vi "Visualizacion_NEW.vi"() -> ()   [LabVIEW 2021] (continued)
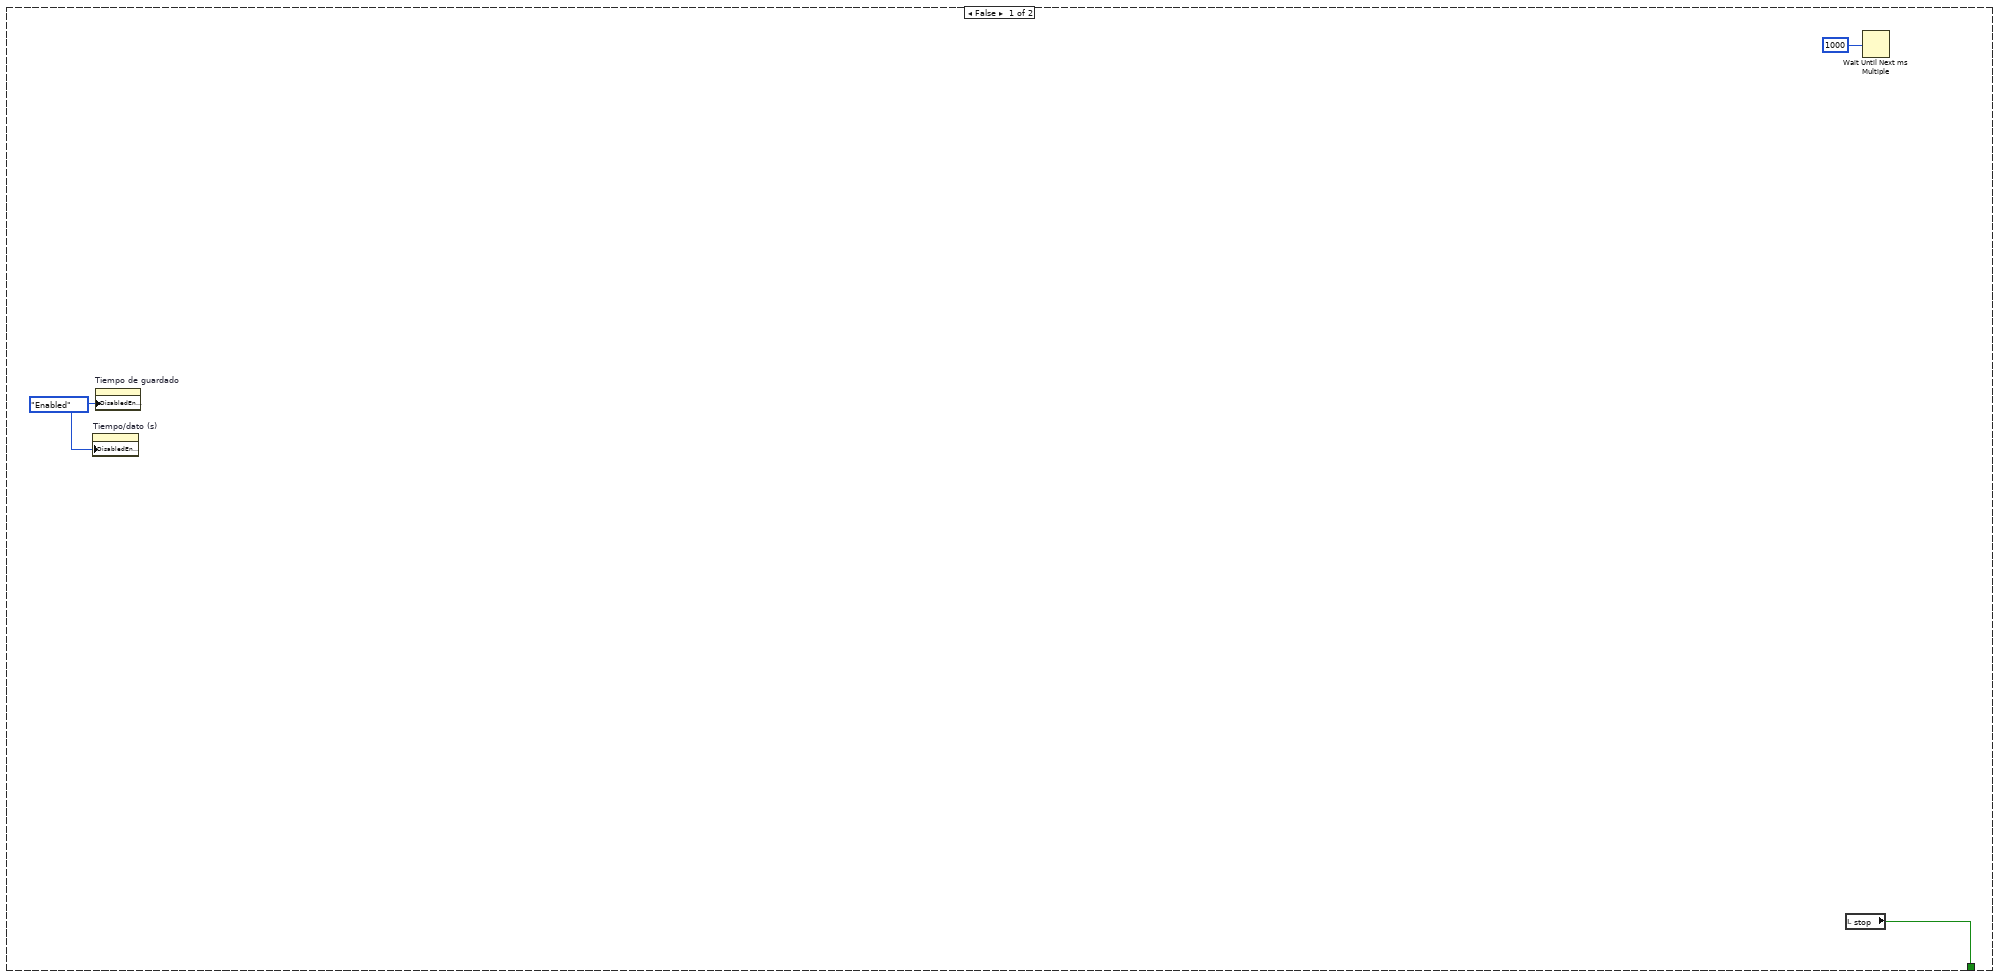
[diagram p2: hidden frame]
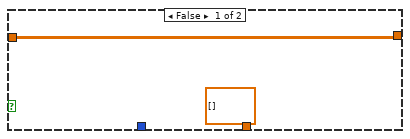
[diagram p3: hidden frame]
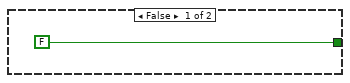
[diagram p4: hidden frame]
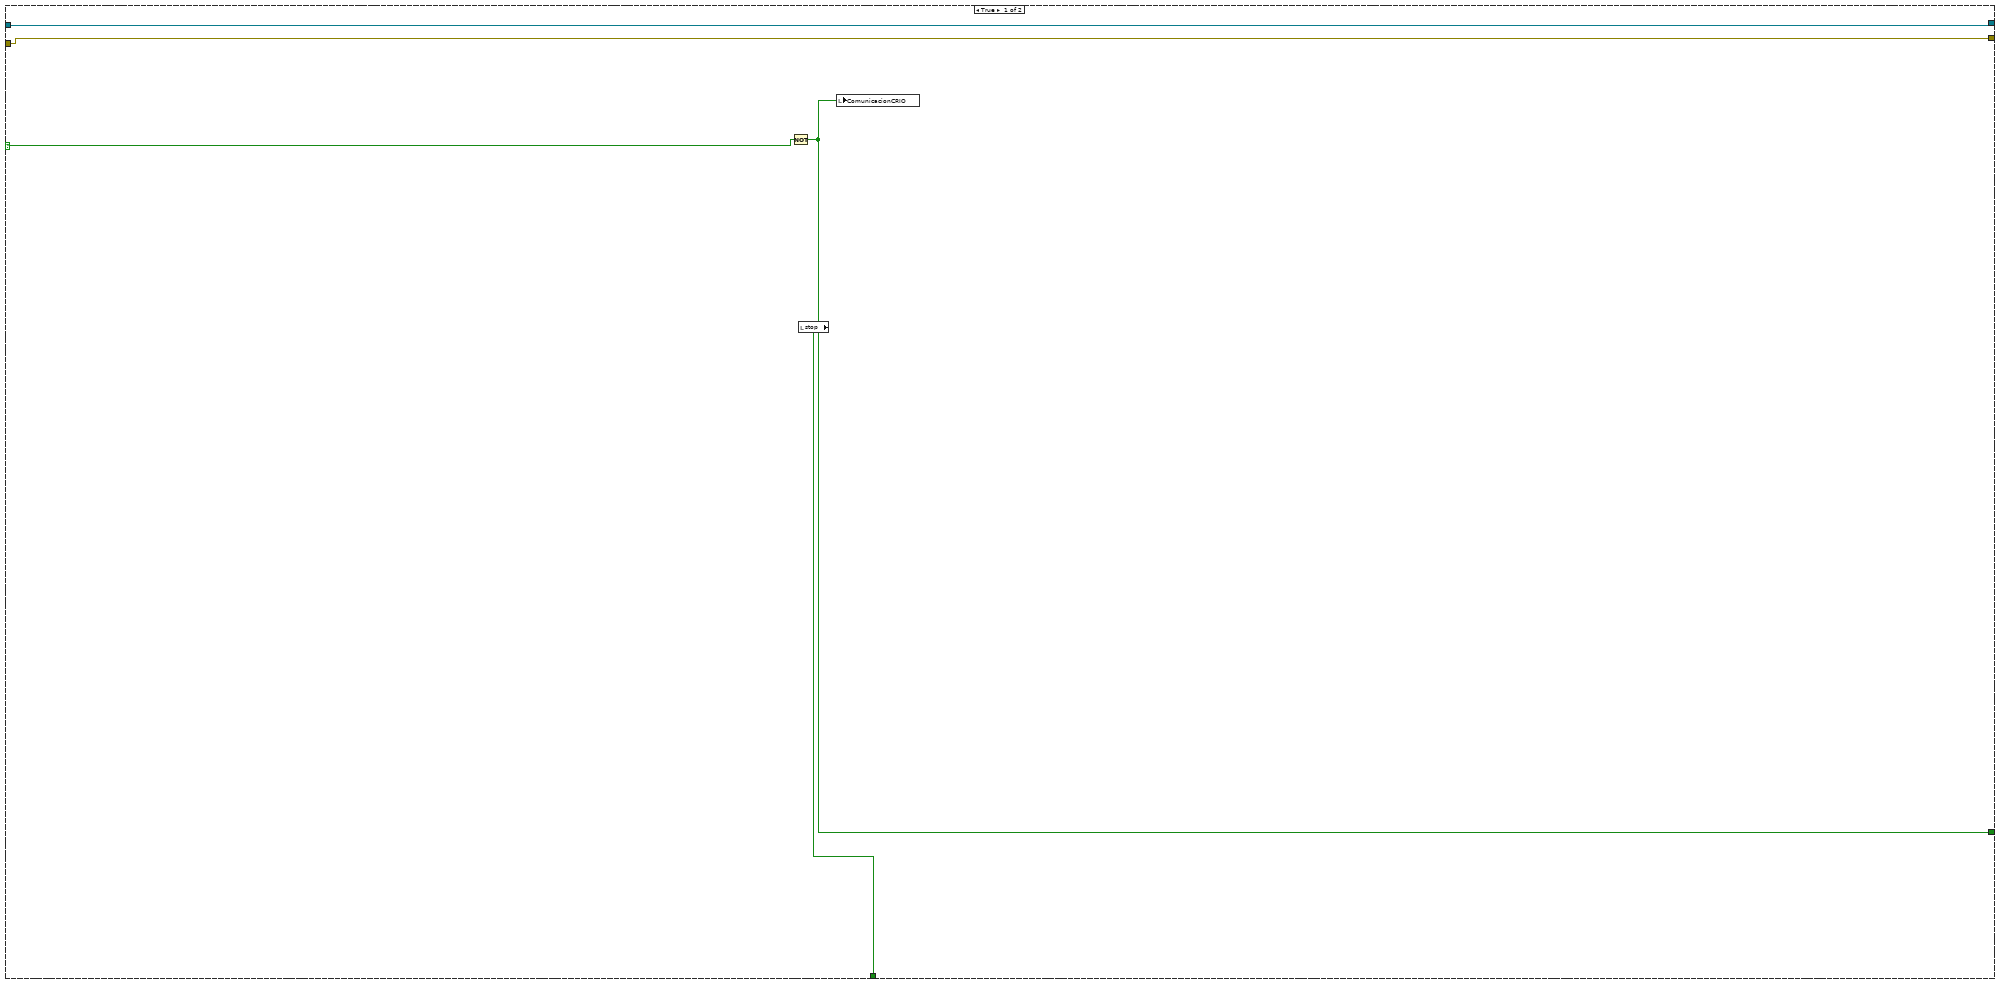
[diagram p6: hidden frame]
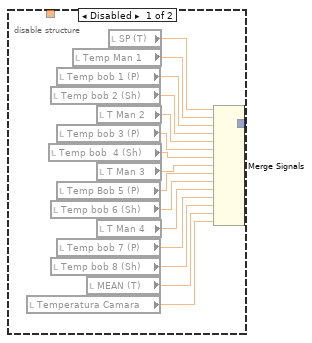
[diagram p12: hidden frame]
                    }
                  }
                }
              }
              n125 = Transpose 2D Array(2D array=w161) -> (transposed array=w160:dbl[][])
              n126 = Multiply(x="Tiempo/dato (s)", y=u32 1000) -> (x*y=w117:u32)
              n127 = Wait Until Next ms Multiple(millisecond multiple=w117) -> ()  [unwired: 1 out]
            }
          }
        }
      }
      n128 = while {
        tunnel: w24 -> [_]
        tunnel: w23 -> [_]
        tunnel: w22 -> [_]
        stop <- w219 stop-if-true
        n129 = flat-sequence {
          tunnel: [w228] -> w222
          tunnel: [w227] -> w221
          tunnel: [w226] -> w220
          tunnel: [w225] -> w219
          tunnel: w222 -> [w442]
          tunnel: w221 -> [w441]
          tunnel: w220 -> [w440]
          frame #0 {
            n130 = call-poly <vilib>:"Create Master Instance.vi"("address"="192.168.111.60") -> ("error out"=w224:errorcluster, "TCP master instance"=w229:refnum<class "Modbus Master.lvclass">)  [unwired: 9 in]
            "Comunicacion Modbus" <- w224
            n131 = Unbundle By Name(w224) -> ("status"=w223:bool)
            n132 = case shown="False" w223 {
              selector: w223 -> [w232 _]
              tunnel: w229 -> [w235 w241]
              tunnel: [w233 w240] -> w228
              tunnel: [w235 w239] -> w227
              tunnel: [w234 w238] -> w226
              tunnel: [w231 w237] -> w225
              tunnel: w224 -> [w234 w236]
              frame True {
                n133 = Not(x=w232) -> (.not. x?=w233:bool)
                n134 = local read "stop"() -> (w231:bool)
                n135 = local write "ComunicacionCRIO"(w233) -> ()
              }
              frame False {
                n136 = while {
                  shift-right: [w290] -> w239
                  shift-left: w241 -> [w340]
                  shift-right: [w289] -> w238
                  shift-left: w236 -> [w339]
                  tunnel: [w336] -> w240
                  tunnel: [w334] -> w237
                  stop <- w338 stop-if-true
                  w248 = u16 0 ("element")
                  w249 = FALSE ("element")
                  # "Para leer variables de fugas"
                  n137 = call-dynamic "Read Coils.vi"("error in (no error)"=w339, "number of coils"=u16 43, "starting address"=u16 1, "Modbus master in"=w340) -> ("error out"=w327:errorcluster, "coil values"=w331:bool[], "Modbus master out"=w328:refnum<class "Modbus Master.lvclass">)  [unwired: 5 in]
                  n138 = local write "coil values"(w331) -> ()
                  n139 = call-dynamic "Read Coils.vi"("error in (no error)"=w327, "number of coils"=u16 1, "starting address"=u16 4, "Modbus master in"=w328) -> ("error out"=w325:errorcluster, "coil values"=w322:bool[], "Modbus master out"=w326:refnum<class "Modbus Master.lvclass">)  [unwired: 5 in]
                  n140 = Index Array(array=w322, index=0) -> (element=→"DO H2 Lab":bool)
                  n141 = call-dynamic "Read Holding Registers.vi"("error in (no error)"=w325, "number of holding registers"=u16 53, "starting address"=u16 100, "Modbus master in"=w326) -> ("error out"=w258:errorcluster, "register values"=w342:u16[], "Modbus master out"=w260:refnum<class "Modbus Master.lvclass">)  [unwired: 5 in]
                  n142 = Split 1D Array(array=w342, index=9) -> (first subarray=w341:u16[], second subarray=w346:u16[])
                  n143 = Array Size(array=w346) -> (size(s)=w345:i32)
                  n144 = Quotient & Remainder(x=w345, y=2) -> (floor(x/y)=w343:i32)  [unwired: 1 out]
                  n145 = for {
                    N: w343 -> [_]
                    tunnel: w346 -> [w432]
                    tunnel: [w429] -> w329 mode=indexing
                    i -> [w439]
                    n146 = Multiply(x=2, y=w439) -> (x*y=w437:i32)
                    n147 = Add(x=w437, y=1) -> (x+y=w435:i32)
                    n148 = Index Array(array=w432, index #1=w437, index #2=w435) -> (element #1=w434:u16, element #2=w433:u16)
                    n149 = Join Numbers(hi=w434, lo=w433) -> ((hi.lo)=w431:u32)
                    n150 = To Single Precision Float(number=w431) -> (single precision float=w428:sgl)
                    n151 = Subtract(x=w428, y=sgl 10000.0) -> (x-y=w426:sgl)
                    n152 = Divide(x=w426, y=sgl 100.0) -> (x/y=w429:sgl)
                  }
                  n153 = for {
                    tunnel: w341 -> [w425] mode=indexing
                    tunnel: [w423] -> w330 mode=indexing
                    n154 = Subtract(x=w425, y=u16 10000) -> (x-y=w423:u16)
                  }
                  n155 = call-dynamic "Read Holding Registers.vi"("error in (no error)"=w258, "number of holding registers"=u16 12, "starting address"=u16 160, "Modbus master in"=w260) -> ("error out"=w257:errorcluster, "register values"=w254:u16[], "Modbus master out"=w259:refnum<class "Modbus Master.lvclass">)  [unwired: 5 in]
                  n156 = for {
                    N: 6 -> [_]
                    tunnel: w254 -> [w358]
                    tunnel: [w354] -> w252 mode=indexing
                    i -> [w365]
                    n157 = Multiply(x=2, y=w365) -> (x*y=w363:i32)
                    n158 = Add(x=w363, y=1) -> (x+y=w361:i32)
                    n159 = Index Array(array=w358, index #1=w363, index #2=w361) -> (element #1=w360:u16, element #2=w359:u16)
                    n160 = Join Numbers(hi=w360, lo=w359) -> ((hi.lo)=w357:u32)
                    n161 = To Single Precision Float(number=w357) -> (single precision float=w352:sgl)
                    n162 = Subtract(x=w352, y=sgl 10000.0) -> (x-y=w355:sgl)
                    n163 = Divide(x=w355, y=sgl 100.0) -> (x/y=w354:sgl)
                  }
                  n164 = local write "Int values"(w330) -> ()
                  n165 = local write "SGL values"(w329) -> ()
                  n166 = local read "Coils write"() -> (w332:bool[])
                  n167 = Index Array(array=w252) -> (element #1=→"USO DE RAM (%)":sgl, element #2=→"USO DE DISCO(%)":sgl, element #3=→"O2":sgl, element #4=→"CO":sgl, element #5=→"LEL":sgl, element #6=→"Contador Ciclos":sgl)  [unwired: 6 in]
                  n168 = call-dynamic "Write Multiple Coils.vi"("error in (no error)"=w257, "coil values"=w332, "starting address"=u16 200, "Modbus master in"=w259) -> ("error out"=w318:errorcluster, "Modbus master out"=w319:refnum<class "Modbus Master.lvclass">)  [unwired: 6 in]
                  n169 = Build Array("Test PID (ºC)") -> (w316:bool[])
                  n170 = call-dynamic "Write Multiple Coils.vi"("error in (no error)"=w318, "coil values"=w316, "starting address"=u16 250, "Modbus master in"=w319) -> ("error out"=w301:errorcluster, "Modbus master out"=w302:refnum<class "Modbus Master.lvclass">)  [unwired: 6 in]
                  n171 = Build Array("Enable PI 1", "Enable PI 2", "Enable PI 3", "Enable PI 4", w249, w249, w249, w249) -> (w303:bool[])
                  n172 = call-dynamic "Write Multiple Coils.vi"("error in (no error)"=w301, "coil values"=w303, "starting address"=u16 240, "Modbus master in"=w302) -> ("error out"=w296:errorcluster, "Modbus master out"=w300:refnum<class "Modbus Master.lvclass">)  [unwired: 6 in]
                  n173 = Build Array("Descarte Media Temps") -> (w298:u16[])
                  n174 = Unbundle By Name(w318) -> ("status"=w337:bool)
                  n175 = call-dynamic "Write Multiple Holding Registers.vi"("error in (no error)"=w296, "holding register values"=w298, "starting address"=u16 350, "Modbus master in"=w300) -> ("error out"=w269:errorcluster, "Modbus master out"=w271:refnum<class "Modbus Master.lvclass">)  [unwired: 6 in]
                  n176 = local read "stop"() -> (w334:bool)
                  n177 = Build Array("SP HR (CC)", "SP Temperatura (CC)") -> (w264:dbl[])
                  n178 = Array Size(array=w264) -> (size(s)=w265:i32)
                  n179 = for {
                    N: w265 -> [_]
                    shift-right: [w367] -> w262
                    shift-left: u16[] [0, 0, 0, 0] -> [w368]
                    tunnel: w264 -> [w366] mode=indexing
                    i -> [w375]
                    n180 = Multiply(x=2, y=w375) -> (x*y=w371:i32)
                    n181 = call "double_2u16.vi"("Entrada"=w366) -> ("Salida 2"=w372:u16, "Salida 1"=w373:u16)  [unwired: 9 in]
                    n182 = Add(x=1, y=w371) -> (x+y=w369:i32)
                    n183 = Replace Array Subset(array=w368, new element #1=w373, index #1=w371, new element #2=w372, index #2=w369) -> (w367:u16[])
                  }
                  n184 = call-dynamic "Write Multiple Holding Registers.vi"("error in (no error)"=w269, "holding register values"=w262, "starting address"=u16 418, "Modbus master in"=w271) -> ("error out"=w268:errorcluster, "Modbus master out"=w270:refnum<class "Modbus Master.lvclass">)  [unwired: 6 in]
                  n185 = Or(x=w337, y=w334) -> (x .or. y?=w338:bool)
                  n186 = Not(x=w337) -> (.not. x?=w336:bool)
                  "ComunicacionCRIO" <- w336
                  n187 = Build Array("TestPID 1(ºC)", "TestPID 2(ºC)", "TestPID3(ºC)", "TestPID 4(ºC)", w248, w248, w248, w248) -> (w313:u16[])
                  n188 = call-dynamic "Write Multiple Holding Registers.vi"("error in (no error)"=w268, "holding register values"=w313, "starting address"=u16 260, "Modbus master in"=w270) -> ("error out"=w281:errorcluster, "Modbus master out"=w280:refnum<class "Modbus Master.lvclass">)  [unwired: 6 in]
                  n189 = local read "Save Parameters"() -> (w273:bool)
                  n190 = local read "DI Sim Bitron Param"() -> (w283:bool)
                  n191 = feedback-in #2(w273) -> ()
                  n192 = feedback #2(w273) -> (w275:bool)
                  n193 = Not(x=w275) -> (.not. x?=w274:bool)
                  n194 = And(x=w273, y=w274) -> (x .and. y?=w272:bool)
                  n195 = case shown="True" w273 {
                    tunnel: w281 -> [w390 w395]
                    tunnel: w280 -> [w391 w396]
                    tunnel: [w391 w396] -> w279
                    tunnel: [w390 w395] -> w278
                    frame False {
                    }
                    frame True {
                      n196 = Build Array("Setpoint corte frío(ºC)", "Setpoint Frío(ºC)", "Setpoint calor cam", "Setpoint calor corte rampa(ºC)", "Setpoint peltiers(ºC)", "Tiempo estabilidad de Frío(min)", "Tiempo mínimo de ciclo(min)", "Tiempo máximo de ciclo(min)", "Cam ºC/min", "Pelt ºC/min", "Tiempo ciclo (Bitron FSM Sim)", "Tiempo Ciclo 0 (min)", "Offset de ciclo.", "trigger bob frio (ºC)") -> (w409:dbl[])
                      n197 = Array Size(array=w409) -> (size(s)=w410:i32)
                      n198 = for {
                        N: w410 -> [_]
                        shift-right: [w414] -> w411
                        shift-left: u16[] [0, 0, 0, 0, 0, 0, 0, 0, 0, 0, 0, 0, 0, 0, 0, 0, 0, 0, 0, 0, 0, 0, 0, 0, 0, 0, 0, 0] -> [w415]
                        tunnel: w409 -> [w413] mode=indexing
                        i -> [w422]
                        n199 = Multiply(x=2, y=w422) -> (x*y=w418:i32)
                        n200 = call "double_2u16.vi"("Entrada"=w413) -> ("Salida 2"=w419:u16, "Salida 1"=w420:u16)  [unwired: 9 in]
                        n201 = Add(x=1, y=w418) -> (x+y=w416:i32)
                        n202 = Replace Array Subset(array=w415, new element #1=w420, index #1=w418, new element #2=w419, index #2=w416) -> (w414:u16[])
                      }
                      "Parameters" <- w411
                      "DI Sim Bitron Param" <- "Digital Input Bitron Simulation"
                    }
                  }
                  n203 = Build Array("Save Parameters", w283) -> (w284:bool[])
                  n204 = call-dynamic "Write Multiple Coils.vi"("error in (no error)"=w278, "coil values"=w284, "starting address"=u16 204, "Modbus master in"=w279) -> ("error out"=w287:errorcluster, "Modbus master out"=w288:refnum<class "Modbus Master.lvclass">)  [unwired: 6 in]
                  n205 = local read "Parameters"() -> (w282:u16[])
                  n206 = call "Elapsed Time"("Reset"=w272) -> ("Time has Elapsed"=w276:bool)  [unwired: 11 in, 7 out]
                  n207 = call-dynamic "Write Multiple Holding Registers.vi"("error in (no error)"=w287, "holding register values"=w282, "starting address"=u16 300, "Modbus master in"=w288) -> ("error out"=w243:errorcluster, "Modbus master out"=w244:refnum<class "Modbus Master.lvclass">)  [unwired: 6 in]
                  n208 = Wait (ms)(milliseconds to wait=u32 200) -> ()  [unwired: 1 out]
                  n209 = case shown="True" w276 {
                    tunnel: w244 -> [_ _]
                    frame False {
                    }
                    frame True {
                      n210 = local write "Save Parameters"(FALSE ("Save Parameters")) -> ()
                    }
                  }
                  n211 = Build Array("Test PWM (%)") -> (w295:bool[])
                  n212 = call-dynamic "Write Multiple Coils.vi"("error in (no error)"=w243, "coil values"=w295, "starting address"=u16 400, "Modbus master in"=w244) -> ("error out"=w291:errorcluster, "Modbus master out"=w292:refnum<class "Modbus Master.lvclass">)  [unwired: 6 in]
                  n213 = case shown="True" "Test PWM (%)" {
                    tunnel: w292 -> [w378 w389]
                    tunnel: w291 -> [w377 w388]
                    tunnel: [w378 w387] -> w290
                    tunnel: [w377 w386] -> w289
                    frame False {
                    }
                    frame True {
                      w379 = u16 0 ("element")
                      n214 = Build Array("PWM 1(SP) 2", "PWM 2(SP) 2", "PWM 3(SP) 2", "PWM 4(SP)", w379, w379, w379, w379) -> (w380:u16[])
                      n215 = call-dynamic "Write Multiple Holding Registers.vi"("error in (no error)"=w388, "holding register values"=w380, "starting address"=u16 410, "Modbus master in"=w389) -> ("error out"=w386:errorcluster, "Modbus master out"=w387:refnum<class "Modbus Master.lvclass">)  [unwired: 6 in]
                    }
                  }
                }
              }
            }
          }
          frame #1 {
            n216 = case shown="True" w442 {
              tunnel: w441 -> [_ w444]
              tunnel: w440 -> [_ w443]
              frame False {
              }
              frame True {
                n217 = call-dynamic "Close.vi"("error in (no error)"=w443, "Modbus master in"=w444) -> ()  [unwired: 9 in, 1 out]
              }
            }
          }
          frame #2 {
            n218 = Tick Count (ms)() -> (millisecond timer value=w445:u32)
            n219 = while {
              tunnel: w445 -> [w451]
              stop <- w447 stop-if-true
              n220 = Tick Count (ms)() -> (millisecond timer value=w452:u32)
              n221 = local read "stop"() -> (w446:bool)
              n222 = Subtract(x=w452, y=w451) -> (x-y=w450:u32)
              n223 = Greater Or Equal?(x=w450, y=u32 5000) -> (x >= y?=w448:bool)
              n224 = Or(x=w448, y=w446) -> (x .or. y?=w447:bool)
            }
          }
        }
      }
      n225 = while {
        tunnel: w21 -> [_]
        stop <- "stop" stop-if-true
        # "MANIFOLD 2 Y BOBINA 3 Y 4"
        # "MANIFOLD 4 Y BOBINA 7 Y 8"
        # "MANIFOLD 3 Y BOBINA 5 Y 6"
        # "FUGA DE GASES"
        # "MANIFOLD 1 Y BOBINA 1 Y 2"
        # "Visualizacion camara climatica"
        # "Control y visualizacion programa principal"
        n226 = local read "SGL values"() -> (w454:sgl[])
        n227 = local read "SGL values"() -> (w542:sgl[])
        n228 = local read "Temperatura Camara"() -> (w464:dbl)
        n229 = local read "Temp bob 2 (Sh)"() -> (w521:sgl)
        n230 = local read "Temp bob 1 (P)"() -> (w463:sgl)
        n231 = local read "Temp Man 1"() -> (w522:sgl)
        n232 = local read "coil values"() -> (w536:bool[])
        n233 = Index Array(array=w454, index #18=21 ("index")) -> (element #1=→"SP (T)":sgl, element #2=→"Temp Man 1" →"T Man 1":sgl, element #3=→"Temp Man 2" →"T Man 2":sgl, element #4=→"Temp Man 3" →"T Man 3":sgl, element #5=→"Temp Man 4" →"T Man 4":sgl, element #6=→"Temp bob 1 (P)" →"T Bob 1":sgl, element #7=→"Temp bob 3 (P)" →"T Bob 3":sgl, element #8=→"Temp Bob 5 (P)" →"T Bob 5":sgl, element #9=→"Temp bob 7 (P)" →"T Bob 7":sgl, element #10=→"Temp bob 2 (Sh)" →"T bob 9":sgl, element #11=→"Temp bob  4 (Sh)" →"T bob 10":sgl, element #12=→"Temp bob 6 (Sh)" →"T bob 11":sgl, element #13=→"Temp bob 8 (Sh)" →"T bob 12":sgl, element #14=→"Ventil 1" →"Ventil 5":sgl, element #15=→"Ventil 2" →"T bob 6":sgl, element #16=→"Ventil 3" →"T bob 7":sgl, element #17=→"Ventil 4" →"T bob 8":sgl, element #18=w480:sgl)  [unwired: 17 in]
        "MEAN (T)" <- w480
        n234 = local read "MEAN (T)"() -> (w465:sgl)
        n235 = local read "SP (T)"() -> (w523:sgl)
        n236 = Index Array(array=w542, index #1=17 ("index")) -> (element #1=w540:sgl, element #2=w539:sgl, element #3=w538:sgl, element #4=w537:sgl)  [unwired: 3 in]
        "Humedad relativa (HR)" <- w540
        "Temperatura Camara" <- w538
        "Setpoint_hum_write" <- w539
        "Setpoint_temp_write" <- w537
        n237 = local read "MEAN (T)"() -> (w482:sgl)
        n238 = Index Array(array=w536, index=1) -> (element=→"Peltiers enable":bool)
        n239 = Merge Signals(w523, w522, w521, w463, w465, w464) -> (→"VALVULA 1  BOBINAS 1 Y 2":dynamicdata)
        n240 = Get Date/Time In Seconds() -> (seconds since 1Jan1904=w544:timestamp)
        "current time" <- w544
        n241 = To Double Precision Float(number=w544) -> (double precision float=w481:dbl)
        n242 = Merge Signals(w540, w538, w539, w537, w482, w481) -> (→"Camara climatica":dynamicdata)
        n243 = local read "Temp bob  4 (Sh)"() -> (w462:sgl)
        n244 = local read "Temperatura Camara"() -> (w460:dbl)
        n245 = local read "Temp bob 3 (P)"() -> (w502:sgl)
        n246 = local read "MEAN (T)"() -> (w461:sgl)
        n247 = local read "T Man 2"() -> (w503:dbl)
        n248 = local read "SP (T)"() -> (w511:sgl)
        n249 = local read "SP (T)"() -> (w501:sgl)
        n250 = local read "Int values"() -> (w520:u16[])
        n251 = Merge Signals(w511, w503, w502, w462, w461, w460) -> (→"VALVULA 2 Y BOBINA 3 Y 4":dynamicdata)
        n252 = Merge Signals(w501, w480) -> (→"TEMPERATURA MEDIA":dynamicdata)
        n253 = Index Array(array=w520) -> (element #1=→"Segmento_temp":u16, element #2=→"PWM 1(SP)":u16, element #3=→"PWM 2(SP)":u16, element #4=→"PWM 3(SP)":u16, element #5=→"PWM 4(SP)":u16)  [unwired: 9 in, 4 out]
        n254 = local read "coil values"() -> (w470:bool[])
        n255 = local read "coil values"() -> (w533:bool[])
        n256 = local read "Temperatura Camara"() -> (w458:dbl)
        n257 = local read "Temp bob 6 (Sh)"() -> (w455:sgl)
        n258 = local read "Temp Bob 5 (P)"() -> (w456:sgl)
        n259 = Index Array(array=w470, index=2) -> (element=→"senal_bitron":bool)
        n260 = local read "T Man 3"() -> (w508:dbl)
        n261 = Index Array(array=w533, index=0) -> ()  [unwired: 1 out]
        n262 = local read "SP (T)"() -> (w509:sgl)
        n263 = local read "coil values"() -> (w514:bool[])
        n264 = local read "MEAN (T)"() -> (w459:sgl)
        n265 = Index Array(array=w470, index #1=42 ("index")) -> (element #1=→"O2":bool, element #2=→"CO":bool, element #3=→"LEL":bool)  [unwired: 2 in]
        n266 = Index Array(array=w514) -> (element=→"Program Status":bool)  [unwired: 1 in]
        n267 = Merge Signals(w509, w508, w456, w455, w459, w458) -> (→"VALVULA 3 Y BOBINA 5 Y 6":dynamicdata)
        n268 = disable-structure shown="Disabled" {
          frame Disabled {
            n269 = property on="PWM 1(SP)" class="DigNum (strict)" props=["Indicator"]() -> ()  [unwired: 2 in, 3 out]
          }
          frame Enabled {
          }
        }
        n270 = Build Array("run_program", "Pause", "Pause_Entrar_camara", "Stop Ensayo") -> (→"Coils write":bool[])
        n271 = local read "Temperatura Camara"() -> (w457:dbl)
        n272 = local read "Temp bob 7 (P)"() -> (w504:sgl)
        n273 = local read "T Man 4"() -> (w505:dbl)
        n274 = local read "Temp bob 8 (Sh)"() -> (w478:sgl)
        n275 = local read "SP (T)"() -> (w506:sgl)
        n276 = local read "MEAN (T)"() -> (w477:sgl)
        n277 = Merge Signals(w506, w505, w504, w478, w477, w457) -> (→"VALVULA 4 Y BOBINA 7 Y 8":dynamicdata)
        n278 = disable-structure shown="Enabled" {
          disable-tunnel: w454 -> [_ w565]
          disable-tunnel: [_ w564] -> w453
          frame Disabled {
            n279 = local read "Temperatura Camara"() -> (w549:dbl)
            n280 = local read "Temp bob  4 (Sh)"() -> (w557:sgl)
            n281 = local read "Temp bob 2 (Sh)"() -> (w547:sgl)
            n282 = local read "Temp bob 6 (Sh)"() -> (w554:sgl)
            n283 = local read "Temp bob 8 (Sh)"() -> (w551:sgl)
            n284 = local read "Temp bob 1 (P)"() -> (w548:sgl)
            n285 = local read "Temp bob 3 (P)"() -> (w558:sgl)
            n286 = local read "Temp Bob 5 (P)"() -> (w555:sgl)
            n287 = local read "Temp bob 7 (P)"() -> (w552:sgl)
            n288 = local read "Temp Man 1"() -> (w560:sgl)
            n289 = local read "MEAN (T)"() -> (w550:sgl)
            n290 = local read "T Man 2"() -> (w559:dbl)
            n291 = local read "T Man 3"() -> (w556:dbl)
            n292 = local read "T Man 4"() -> (w553:dbl)
            n293 = local read "SP (T)"() -> (w561:sgl)
            n294 = Merge Signals(w561, w560, w548, w547, w559, w558, w557, w556, w555, w554, w553, w552, w551, w550, w549) -> ()  [unwired: 1 out]
          }
          frame Enabled {
            n295 = local read "Temperatura Camara"() -> (w562:dbl)
            n296 = local read "MEAN (T)"() -> (w563:sgl)
            n297 = Index Array(array=w565) -> (element #1=w582:sgl, element #2=w581:sgl, element #3=w580:sgl, element #4=w579:sgl, element #5=w578:sgl, element #6=w577:sgl, element #7=w576:sgl, element #8=w575:sgl, element #9=w574:sgl, element #10=w573:sgl, element #11=w572:sgl, element #12=w571:sgl, element #13=w570:sgl, element #14=w569:sgl, element #15=w568:sgl, element #16=w567:sgl, element #17=w566:sgl)  [unwired: 17 in]
            n298 = Merge Signals(w582, w581, w580, w579, w578, w577, w576, w575, w574, w573, w572, w571, w570, w569, w568, w567, w566, w563, w562) -> (w564:dynamicdata)
          }
        }
        "ALL TOGETHER" <- w453
        n299 = local read "O2"() -> (w474:sgl)
        n300 = local read "CO"() -> (w473:sgl)
        n301 = local read "LEL"() -> (w472:sgl)
        n302 = local read "USO DE DISCO(%)"() -> (→"DISK":sgl)
        n303 = local read "USO DE RAM (%)"() -> (→"RAM":sgl)
        n304 = Merge Signals(w474, w473, w472) -> (→"O2/CO/LEL":dynamicdata)
        n305 = Wait (ms)(milliseconds to wait=u32 500) -> ()  [unwired: 1 out]
      }
      n306 = while {
        stop <- w59 stop-if-true
        # "length array->"
        # "registro ini->"
        # "IMPORTANTE: LOS ARRAYS CUENTAN UNO MENOS QUE LOS REGISTROS"
        n307 = local read "warnings table"() -> (w62:T3)
        n308 = local read "coil values"() -> (w54:bool[])
        n309 = Array Subset(array=w54, index=4, length=19) -> (w51:bool[])
        n310 = call "Historical Warnings (SubVI).vi"("Warnings bool array"=w51, "in"="Reset", "warnings table in"=w62) -> ("Warnings table out"=→"warnings table":T3)  [unwired: 8 in]
        n311 = Array Subset(array=w54, index=23, length=16) -> (w41:bool[])
        n312 = Index Array(array=w54, index #1=20 ("index")) -> (element #1=w50:bool, element #2=w49:bool, element #3=w48:bool)  [unwired: 2 in]
        "W2" <- w50
        "W3" <- w49
        "W4" <- w48
        n313 = Array Subset(array=w54, index=4, length=16) -> (w47:bool[])
        n314 = Build Array (concatenate)(w51, w50, w49, w48, w47) -> (w46:bool[])
        n315 = Index Array(array=w47) -> (element #1=→"W1.1":bool, element #2=→"W1.2":bool, element #3=→"W1.3":bool, element #4=→"W1.4":bool, element #5=→"W1.5":bool, element #6=→"W1.6":bool, element #7=→"W1.7":bool, element #8=→"W1.8":bool, element #9=→"W1.9":bool, element #10=→"W1.10":bool, element #11=→"W1.11":bool, element #12=→"W1.14":bool, element #13=→"W1.12":bool, element #14=→"W1.13":bool, element #15=→"W1.15":bool, element #16=→"W1.16":bool)  [unwired: 16 in]
        n316 = for {
          tunnel: w41 -> [w85] mode=indexing
          shift-right: [w84] -> w43
          shift-left: FALSE -> [w86]
          n317 = Or(x=w85, y=w86) -> (x .or. y?=w84:bool)
        }
        "Error" <- w43
        n318 = for {
          tunnel: w46 -> [w88] mode=indexing
          shift-right: [w87] -> w44
          shift-left: FALSE -> [w89]
          n319 = Or(x=w88, y=w89) -> (x .or. y?=w87:bool)
        }
        "Warning" <- w44
        n320 = local read "W to save"() -> (w55:string[][])
        n321 = call "Saving_Warnings(SubVI).vi"("Warnings bool array"=w51, "Reset"="Warning saved", "W In"=w55) -> ("W Out"=→"W to save":string[][])  [unwired: 8 in]
        n322 = Wait (ms)(milliseconds to wait=u32 20) -> ()  [unwired: 1 out]
        n323 = local read "stop"() -> (w59:bool)
      }
    }
    frame #2 {
      n324 = local write "stop"(w583) -> ()
    }
  }
